vi "Dresden R2R Sputter 03.02.2018 IY24.vi"() -> ()   [LabVIEW 2009] (continued)
                                }
                                }
                                }
                                }
                                }
                                frame #1 {
                                }
                                }
                                }
                                frame #1 {
                                }
                                }
                                }
                                }
                                }
                                frame #1 {
                                }
                                }
                                }
                                frame #1 {
                                n26473 = local read "Semi"() -> (w31686:bool)
                                n26474 = case shown="False" w31686 {
                                frame #0 {
                                n26475 = Wait (ms)(milliseconds to wait=u32 1000) -> ()  [unwired: 1 out]
                                n26476 = local write "SDC1 29"(TRUE ("SDC1 29")) -> ()
                                }
                                frame #1 {
                                }
                                }
                                }
                                }
                                }
                                frame #27 {
                                n26477 = local read "Semi"() -> (w31689:bool)
                                n26478 = case shown="False" w31689 {
                                frame #0 {
                                n26479 = local write "Cnt_Do_Buzzer"(TRUE ("SDC1 30")) -> ()
                                n26480 = Wait (ms)(milliseconds to wait=u32 2500) -> ()  [unwired: 1 out]
                                n26481 = local write "SDC1 30"(TRUE ("SDC1 30")) -> ()
                                }
                                frame #1 {
                                }
                                }
                                }
                                frame #28 {
                                n26482 = local read "Semi"() -> (w31693:bool)
                                n26483 = case shown="False" w31693 {
                                frame #0 {
                                n26484 = local write "Cnt_Do_Buzzer"(FALSE ("SDC1 30")) -> ()
                                n26485 = Wait (ms)(milliseconds to wait=u32 1000) -> ()  [unwired: 1 out]
                                }
                                frame #1 {
                                }
                                }
                                }
                                }
                                }
                                frame #1 {
                                }
                                }
                                }
                              }
                            }
                            frame #1 {
                              n26486 = local read "Single_ch3_Interlock"() -> (w31696:dbl)
                              n26487 = local read "Ch3_pressure"() -> (w31700:dbl)
                              n26488 = local read "started_up_ch3"() -> (w31698:bool)
                              n26489 = In Range and Coerce(upper limit=w31696, x=w31700, lower limit=1e-08) -> (In Range?=w31701:bool)  [unwired: 1 out]
                              n26490 = And(x=w31701, y=w31698) -> (x .and. y?=w31697:bool)
                              n26491 = case shown="True" w31697 {
                                frame #0 {
                                }
                                frame #1 {
                                n26492 = local read "Semi"() -> (w31702:bool)
                                n26493 = case shown="False" w31702 {
                                frame #0 {
                                n26494 = stacked-sequence {
                                frame #0 {
                                n26495 = stacked-sequence {
                                frame #0 {
                                n26496 = local read "Semi"() -> (w31703:bool)
                                n26497 = case shown="False" w31703 {
                                frame #0 {
                                w31707 = FALSE ("Casette_servo_start/stop_do")
                                n26498 = local write "Ch3_Sov_Ar_do"(FALSE ("Ch1_Sov_Ar_do")) -> ()
                                n26499 = local write "Ar_auto_set_zero_ch3"(TRUE ("Dc_auto_set_zero")) -> ()
                                n26500 = local write "Dc_host_auto"(TRUE ("Dc_host_auto")) -> ()
                                n26501 = local write "final_process_messages"("Coating was Completed" ("final_process_messages")) -> ()
                                n26502 = local write "system_status"("Coating Mode is Active" ("system_status")) -> ()
                                n26503 = local write "Casette_servo_start/stop_do"(w31707) -> ()
                                n26504 = local write "Tension_controllers_start/stop_do"(w31707) -> ()
                                n26505 = local write "Cnt_Dcps_sw1_do"(FALSE ("Cnt_Dcps_sw1_do")) -> ()
                                }
                                frame #1 {
                                }
                                }
                                }
                                frame #1 {
                                n26506 = local read "Semi"() -> (w31711:bool)
                                n26507 = case shown="False" w31711 {
                                frame #0 {
                                n26508 = Wait (ms)(milliseconds to wait=u32 2500) -> ()  [unwired: 1 out]
                                }
                                frame #1 {
                                }
                                }
                                }
                                frame #2 {
                                n26509 = local read "Semi"() -> (w31713:bool)
                                n26510 = case shown="False" w31713 {
                                frame #0 {
                                n26511 = local write "Ch2_SRV_start_stop_do"(FALSE ("Ch1_SRV_start_stop_do")) -> ()
                                }
                                frame #1 {
                                }
                                }
                                }
                                frame #3 {
                                n26512 = local read "Semi"() -> (w31715:bool)
                                n26513 = case shown="False" w31715 {
                                frame #0 {
                                n26514 = Wait (ms)(milliseconds to wait=u32 2500) -> ()  [unwired: 1 out]
                                }
                                frame #1 {
                                }
                                }
                                }
                                frame #4 {
                                n26515 = local read "Semi"() -> (w31717:bool)
                                n26516 = case shown="False" w31717 {
                                frame #0 {
                                n26517 = Wait (ms)(milliseconds to wait=u32 1000) -> ()  [unwired: 1 out]
                                n26518 = local write "SDC1 1"(TRUE ("CMW1")) -> ()
                                }
                                frame #1 {
                                }
                                }
                                }
                                }
                                }
                                frame #1 {
                                n26519 = local read "ch_present_position"() -> (w31722:dbl)
                                n26520 = Not Equal?(x=w31722, y=3.0) -> (x != y?=w31720:bool)
                                n26521 = case shown="True" w31720 {
                                frame #0 {
                                }
                                frame #1 {
                                n26522 = stacked-sequence {
                                frame #0 {
                                n26523 = local write "Set chamber"(3.0 ("Set chamber")) -> ()
                                n26524 = Wait (ms)(milliseconds to wait=u32 100) -> ()  [unwired: 1 out]
                                }
                                frame #1 {
                                n26525 = local write "Auto_set_transfer"(TRUE ("Auto_set_transfer")) -> ()
                                }
                                frame #2 {
                                n26526 = while {
                                stop <- w31727 stop-if-true
                                n26527 = Wait Until Next ms Multiple(millisecond multiple=u32 300) -> ()  [unwired: 1 out]
                                n26528 = local read "Auto_set_transfer"() -> (w31728:bool)
                                n26529 = local read "Semi"() -> (w31730:bool)
                                n26530 = Not(x=w31728) -> (.not. x?=w31729:bool)
                                n26531 = Or(x=w31729, y=w31730) -> (x .or. y?=w31727:bool)
                                }
                                }
                                frame #3 {
                                n26532 = Wait (ms)(milliseconds to wait=u32 300) -> ()  [unwired: 1 out]
                                n26533 = local write "SDC2 19"(TRUE ("SMW1 2")) -> ()
                                }
                                }
                                }
                                }
                                }
                                frame #2 {
                                # "WATER FLOW CONTROL OPEN"
                                n26534 = stacked-sequence {
                                frame #0 {
                                n26535 = local read "Semi"() -> (w31733:bool)
                                n26536 = case shown="False" w31733 {
                                frame #0 {
                                n26537 = while {
                                i -> [w31739]
                                stop <- w31734 stop-if-true
                                n26538 = Greater?(x=w31739, y=100) -> (0:w31738:bool)
                                n26539 = case shown="True" w31738 {
                                frame #0 {
                                }
                                frame #1 {
                                n26540 = local write "Semi"(TRUE ("Semi")) -> ()
                                n26541 = local write "Error Message"("Coating Process  \nwas cancelled.\nPlease check water \nflow connection." ("Error Message")) -> ()
                                }
                                }
                                n26542 = local read "Ch4_WFS_di"() -> (w31737:bool)
                                n26543 = case shown="True" w31737 {
                                tunnel: [TRUE FALSE] -> w31736
                                frame #0 {
                                }
                                frame #1 {
                                n26544 = local write "Ch4_WFC_do"(FALSE ("Ch1_WFC_do")) -> ()
                                n26545 = Wait Until Next ms Multiple(millisecond multiple=u32 200) -> ()  [unwired: 1 out]
                                }
                                }
                                n26546 = local read "Semi"() -> (w31735:bool)
                                n26547 = Or(x=w31736, y=w31735) -> (x .or. y?=w31734:bool)
                                }
                                }
                                frame #1 {
                                }
                                }
                                }
                                frame #1 {
                                n26548 = local read "Semi"() -> (w31747:bool)
                                n26549 = case shown="False" w31747 {
                                frame #0 {
                                n26550 = while {
                                i -> [w31753]
                                stop <- w31748 stop-if-true
                                n26551 = Greater?(x=w31753, y=100) -> (0:w31752:bool)
                                n26552 = case shown="True" w31752 {
                                frame #0 {
                                }
                                frame #1 {
                                n26553 = local write "Semi"(TRUE ("Semi")) -> ()
                                n26554 = local write "Error Message"("Coating Process  \nwas cancelled.\nPlease check water \nflow connection." ("Error Message")) -> ()
                                }
                                }
                                n26555 = local read "Ch1_WFS_di"() -> (w31751:bool)
                                n26556 = case shown="True" w31751 {
                                tunnel: [TRUE FALSE] -> w31750
                                frame #0 {
                                }
                                frame #1 {
                                n26557 = local write "Ch1_WFC_do"(FALSE ("Ch1_WFC_do")) -> ()
                                n26558 = Wait Until Next ms Multiple(millisecond multiple=u32 200) -> ()  [unwired: 1 out]
                                }
                                }
                                n26559 = local read "Semi"() -> (w31749:bool)
                                n26560 = Or(x=w31750, y=w31749) -> (x .or. y?=w31748:bool)
                                }
                                }
                                frame #1 {
                                }
                                }
                                }
                                frame #2 {
                                n26561 = local read "Semi"() -> (w31761:bool)
                                n26562 = case shown="False" w31761 {
                                frame #0 {
                                n26563 = while {
                                i -> [w31767]
                                stop <- w31762 stop-if-true
                                n26564 = Greater?(x=w31767, y=100) -> (0:w31766:bool)
                                n26565 = case shown="True" w31766 {
                                frame #0 {
                                }
                                frame #1 {
                                n26566 = local write "Semi"(TRUE ("Semi")) -> ()
                                n26567 = local write "Error Message"("Coating Process  \nwas cancelled.\nPlease check water \nflow connection." ("Error Message")) -> ()
                                }
                                }
                                n26568 = local read "Ch2_WFS_di"() -> (w31765:bool)
                                n26569 = case shown="True" w31765 {
                                tunnel: [TRUE FALSE] -> w31764
                                frame #0 {
                                }
                                frame #1 {
                                n26570 = local write "Ch2_WFC_do"(FALSE ("Ch1_WFC_do")) -> ()
                                n26571 = Wait Until Next ms Multiple(millisecond multiple=u32 200) -> ()  [unwired: 1 out]
                                }
                                }
                                n26572 = local read "Semi"() -> (w31763:bool)
                                n26573 = Or(x=w31764, y=w31763) -> (x .or. y?=w31762:bool)
                                }
                                }
                                frame #1 {
                                }
                                }
                                }
                                frame #3 {
                                n26574 = local read "Semi"() -> (w31775:bool)
                                n26575 = case shown="False" w31775 {
                                frame #0 {
                                n26576 = local write "SDC1 2"(TRUE ("SDC1 2")) -> ()
                                n26577 = Wait (ms)(milliseconds to wait=u32 1000) -> ()  [unwired: 1 out]
                                }
                                frame #1 {
                                }
                                }
                                }
                                frame #4 {
                                n26578 = local read "Semi"() -> (w31778:bool)
                                n26579 = case shown="False" w31778 {
                                frame #0 {
                                n26580 = while {
                                i -> [w31784]
                                stop <- w31779 stop-if-true
                                n26581 = Greater?(x=w31784, y=100) -> (0:w31783:bool)
                                n26582 = case shown="True" w31783 {
                                frame #0 {
                                }
                                frame #1 {
                                n26583 = local write "Semi"(TRUE ("Semi")) -> ()
                                n26584 = local write "Error Message"("Coating Process  \nwas cancelled.\nPlease check water \nflow connection." ("Error Message")) -> ()
                                }
                                }
                                n26585 = local read "Ch3_WFS_di"() -> (w31782:bool)
                                n26586 = case shown="False" w31782 {
                                tunnel: [FALSE TRUE] -> w31781
                                frame #0 {
                                n26587 = local write "Ch3_WFC_do"(TRUE ("Ch1_WFC_do")) -> ()
                                n26588 = Wait Until Next ms Multiple(millisecond multiple=u32 200) -> ()  [unwired: 1 out]
                                }
                                frame #1 {
                                }
                                }
                                n26589 = local read "Semi"() -> (w31780:bool)
                                n26590 = Or(x=w31781, y=w31780) -> (x .or. y?=w31779:bool)
                                }
                                }
                                frame #1 {
                                }
                                }
                                }
                                }
                                }
                                frame #3 {
                                # "BG-BV open"
                                n26591 = stacked-sequence {
                                frame #0 {
                                n26592 = local read "Semi"() -> (w31792:bool)
                                n26593 = case shown="False" w31792 {
                                frame #0 {
                                n26594 = while {
                                i -> [w31798]
                                stop <- w31793 stop-if-true
                                n26595 = Greater?(x=w31798, y=50) -> (0:w31797:bool)
                                n26596 = case shown="True" w31797 {
                                frame #0 {
                                }
                                frame #1 {
                                n26597 = local write "Semi"(TRUE ("Semi")) -> ()
                                n26598 = local write "Error Message"("Coating Process  \nwas cancelled.\nPlease check \nBG-BV connection." ("Error Message")) -> ()
                                }
                                }
                                n26599 = local read "Ch3_Bg_bv_di"() -> (w31796:bool)
                                n26600 = case shown="False" w31796 {
                                tunnel: [FALSE TRUE] -> w31795
                                frame #0 {
                                n26601 = local write "Ch3_Bg_bv_do"(TRUE ("Ch1_WFC_do")) -> ()
                                n26602 = Wait Until Next ms Multiple(millisecond multiple=u32 200) -> ()  [unwired: 1 out]
                                }
                                frame #1 {
                                }
                                }
                                n26603 = local read "Semi"() -> (w31794:bool)
                                n26604 = Or(x=w31795, y=w31794) -> (x .or. y?=w31793:bool)
                                }
                                }
                                frame #1 {
                                }
                                }
                                }
                                frame #1 {
                                n26605 = local read "Semi"() -> (w31806:bool)
                                n26606 = case shown="False" w31806 {
                                frame #0 {
                                n26607 = Wait (ms)(milliseconds to wait=u32 1000) -> ()  [unwired: 1 out]
                                n26608 = local write "SDC1 4"(TRUE ("SDC1 4")) -> ()
                                }
                                frame #1 {
                                }
                                }
                                }
                                }
                                }
                                frame #4 {
                                # "Baratron set zero"
                                n26609 = stacked-sequence {
                                frame #0 {
                                n26610 = local write "Pc_bv3_auto_baratron_set_zero"(TRUE ("Pc_bv2_auto_baratron_set_zero")) -> ()
                                }
                                frame #1 {
                                n26611 = while {
                                i -> [w31814]
                                stop <- w31811 stop-if-true
                                n26612 = Greater?(x=w31814, y=50 ("Baratron set zero time 2")) -> (0:w31813:bool)
                                n26613 = case shown="True" w31813 {
                                frame #0 {
                                }
                                frame #1 {
                                n26614 = local write "Semi"(TRUE ("Semi")) -> ()
                                n26615 = local write "Error Message"("" ("Error Message")) -> ()
                                }
                                }
                                n26616 = local read "Pressure_ch3"() -> (w31810:i32)
                                n26617 = Less?(x=w31810, y=0.1 ("Pressure Check for baratron set zero")) -> (x < y?=w31817:bool)
                                n26618 = case shown="False" w31817 {
                                tunnel: [FALSE TRUE] -> w31816
                                frame #0 {
                                n26619 = Wait Until Next ms Multiple(millisecond multiple=u32 200) -> ()  [unwired: 1 out]
                                }
                                frame #1 {
                                }
                                }
                                n26620 = local read "Semi"() -> (w31815:bool)
                                n26621 = Or(x=w31816, y=w31815) -> (x .or. y?=w31811:bool)
                                }
                                }
                                frame #2 {
                                n26622 = local read "Semi"() -> (w31824:bool)
                                n26623 = case shown="False" w31824 {
                                frame #0 {
                                n26624 = local write "SDC1 2b"(TRUE ("SDC1 2b")) -> ()
                                n26625 = Wait (ms)(milliseconds to wait=u32 1000) -> ()  [unwired: 1 out]
                                }
                                frame #1 {
                                }
                                }
                                }
                                }
                                }
                                frame #5 {
                                # "CC CLOSE"
                                n26626 = stacked-sequence {
                                frame #0 {
                                n26627 = local read "Semi"() -> (w31827:bool)
                                n26628 = case shown="False" w31827 {
                                frame #0 {
                                n26629 = while {
                                i -> [w31833]
                                stop <- w31828 stop-if-true
                                n26630 = Greater?(x=w31833, y=50) -> (0:w31832:bool)
                                n26631 = case shown="True" w31832 {
                                frame #0 {
                                }
                                frame #1 {
                                n26632 = local write "Semi"(TRUE ("Semi")) -> ()
                                n26633 = local write "Error Message"("Coating Process  \nwas cancelled.\nPlease check \nBG-BV connection." ("Error Message")) -> ()
                                }
                                }
                                n26634 = local read "Ch3_Cc_on_off_di"() -> (w31831:bool)
                                n26635 = case shown="True" w31831 {
                                tunnel: [TRUE FALSE] -> w31830
                                frame #0 {
                                }
                                frame #1 {
                                n26636 = local write "Ch3_Cc_on_off_do"(FALSE ("Ch1_WFC_do")) -> ()
                                n26637 = Wait Until Next ms Multiple(millisecond multiple=u32 200) -> ()  [unwired: 1 out]
                                }
                                }
                                n26638 = local read "Semi"() -> (w31829:bool)
                                n26639 = Or(x=w31830, y=w31829) -> (x .or. y?=w31828:bool)
                                }
                                }
                                frame #1 {
                                }
                                }
                                }
                                frame #1 {
                                n26640 = local read "Semi"() -> (w31841:bool)
                                n26641 = case shown="False" w31841 {
                                frame #0 {
                                n26642 = local write "SDC1 3"(TRUE ("SDC1 3")) -> ()
                                n26643 = Wait (ms)(milliseconds to wait=u32 1000) -> ()  [unwired: 1 out]
                                }
                                frame #1 {
                                }
                                }
                                }
                                }
                                }
                                frame #6 {
                                # "PC-BV CLOSE"
                                n26644 = stacked-sequence {
                                frame #0 {
                                n26645 = local read "Semi"() -> (w31844:bool)
                                n26646 = case shown="False" w31844 {
                                frame #0 {
                                n26647 = stacked-sequence {
                                frame #0 {
                                n26648 = local read "Semi"() -> (w31845:bool)
                                n26649 = case shown="False" w31845 {
                                frame #0 {
                                n26650 = local write "Pc_bv3_auto_close"(TRUE ("Tp1_auto_start")) -> ()
                                }
                                frame #1 {
                                }
                                }
                                }
                                frame #1 {
                                n26651 = local read "Semi"() -> (w31847:bool)
                                n26652 = case shown="False" w31847 {
                                frame #0 {
                                n26653 = Wait (ms)(milliseconds to wait=u32 1000) -> ()  [unwired: 1 out]
                                }
                                frame #1 {
                                }
                                }
                                }
                                frame #2 {
                                n26654 = local read "Semi"() -> (w31849:bool)
                                n26655 = case shown="False" w31849 {
                                frame #0 {
                                n26656 = while {
                                i -> [w31855]
                                stop <- w31851 stop-if-true
                                n26657 = local read "Pc_bv_closed_ch3"() -> (w31853:bool)
                                n26658 = Greater?(x=w31855, y=120) -> (0:w31854:bool)
                                n26659 = local read "Semi"() -> (w31852:bool)
                                n26660 = Compound Arithmetic op=OR(w31852, w31853, w31854) -> (w31851:bool)
                                n26661 = Wait (ms)(milliseconds to wait=u32 500) -> ()  [unwired: 1 out]
                                }
                                }
                                frame #1 {
                                }
                                }
                                }
                                frame #3 {
                                n26662 = local read "Semi"() -> (w31857:bool)
                                n26663 = case shown="False" w31857 {
                                frame #0 {
                                n26664 = local read "Pc_bv_closed_ch3"() -> (w31858:bool)
                                n26665 = case shown="False" w31858 {
                                frame #0 {
                                n26666 = local write "Pc_bv3_auto_close"(TRUE ("Pc_bv1_auto_open")) -> ()
                                }
                                frame #1 {
                                }
                                }
                                }
                                frame #1 {
                                }
                                }
                                }
                                frame #4 {
                                n26667 = local read "Semi"() -> (w31860:bool)
                                n26668 = case shown="False" w31860 {
                                frame #0 {
                                n26669 = local read "Pc_bv_closed_ch3"() -> (w31861:bool)
                                n26670 = case shown="False" w31861 {
                                frame #0 {
                                n26671 = Wait (ms)(milliseconds to wait=u32 1000) -> ()  [unwired: 1 out]
                                }
                                frame #1 {
                                }
                                }
                                }
                                frame #1 {
                                }
                                }
                                }
                                frame #5 {
                                n26672 = local read "Semi"() -> (w31863:bool)
                                n26673 = case shown="False" w31863 {
                                frame #0 {
                                n26674 = while {
                                i -> [w31869]
                                stop <- w31865 stop-if-true
                                n26675 = local read "Pc_bv_closed_ch3"() -> (w31867:bool)
                                n26676 = Greater?(x=w31869, y=120) -> (0:w31868:bool)
                                n26677 = local read "Semi"() -> (w31866:bool)
                                n26678 = Compound Arithmetic op=OR(w31866, w31867, w31868) -> (w31865:bool)
                                n26679 = Wait (ms)(milliseconds to wait=u32 500) -> ()  [unwired: 1 out]
                                }
                                }
                                frame #1 {
                                }
                                }
                                }
                                frame #6 {
                                n26680 = local read "Semi"() -> (w31871:bool)
                                n26681 = case shown="False" w31871 {
                                frame #0 {
                                n26682 = local read "Pc_bv_closed_ch3"() -> (w31872:bool)
                                n26683 = case shown="False" w31872 {
                                frame #0 {
                                n26684 = local write "Error Message"("Start up process  cancelled\nbecause  PC-BV not closed.\nPlease check PC-BV1 connections." ("Error Message")) -> ()
                                n26685 = Wait (ms)(milliseconds to wait=u32 1000) -> ()  [unwired: 1 out]
                                }
                                frame #1 {
                                }
                                }
                                }
                                frame #1 {
                                }
                                }
                                }
                                }
                                }
                                frame #1 {
                                }
                                }
                                }
                                frame #1 {
                                n26686 = local read "Semi"() -> (w31875:bool)
                                n26687 = case shown="False" w31875 {
                                frame #0 {
                                n26688 = local write "SDC1 5"(TRUE ("SDC1 5")) -> ()
                                n26689 = Wait (ms)(milliseconds to wait=u32 1000) -> ()  [unwired: 1 out]
                                }
                                frame #1 {
                                }
                                }
                                }
                                }
                                }
                                frame #7 {
                                # "SOV-AR OPEN"
                                n26690 = stacked-sequence {
                                frame #0 {
                                n26691 = local read "Semi"() -> (w31878:bool)
                                n26692 = case shown="False" w31878 {
                                frame #0 {
                                n26693 = while {
                                i -> [w31884]
                                stop <- w31879 stop-if-true
                                n26694 = Greater?(x=w31884, y=50) -> (0:w31883:bool)
                                n26695 = case shown="True" w31883 {
                                frame #0 {
                                }
                                frame #1 {
                                n26696 = local write "Semi"(TRUE ("Semi")) -> ()
                                n26697 = local write "Error Message"("Coating Process  \nwas cancelled.\nPlease check \nSOV-Ar connection." ("Error Message")) -> ()
                                }
                                }
                                n26698 = local read "Ch3_Sov_Ar_di"() -> (w31882:bool)
                                n26699 = case shown="False" w31882 {
                                tunnel: [FALSE TRUE] -> w31881
                                frame #0 {
                                n26700 = local write "Ch3_Sov_Ar_do"(TRUE ("Ch1_WFC_do")) -> ()
                                n26701 = Wait Until Next ms Multiple(millisecond multiple=u32 200) -> ()  [unwired: 1 out]
                                }
                                frame #1 {
                                }
                                }
                                n26702 = local read "Semi"() -> (w31880:bool)
                                n26703 = Or(x=w31881, y=w31880) -> (x .or. y?=w31879:bool)
                                }
                                }
                                frame #1 {
                                }
                                }
                                }
                                frame #1 {
                                n26704 = local read "Semi"() -> (w31892:bool)
                                n26705 = case shown="False" w31892 {
                                frame #0 {
                                n26706 = while {
                                i -> [w31897]
                                stop <- w31895 stop-if-true
                                n26707 = Greater?(x=w31897, y=5) -> (0:w31893:bool)
                                n26708 = Wait Until Next ms Multiple(millisecond multiple=u32 1000) -> ()  [unwired: 1 out]
                                n26709 = local read "Semi"() -> (w31896:bool)
                                n26710 = Or(x=w31893, y=w31896) -> (x .or. y?=w31895:bool)
                                }
                                }
                                frame #1 {
                                }
                                }
                                }
                                frame #2 {
                                n26711 = local read "Semi"() -> (w31899:bool)
                                n26712 = case shown="False" w31899 {
                                frame #0 {
                                n26713 = local write "SDC1 6"(TRUE ("SDC1 6")) -> ()
                                n26714 = Wait (ms)(milliseconds to wait=u32 1000) -> ()  [unwired: 1 out]
                                }
                                frame #1 {
                                }
                                }
                                }
                                }
                                }
                                frame #8 {
                                # "CHECK CHAMBER PRESSURE"
                                n26715 = stacked-sequence {
                                frame #0 {
                                n26716 = local read "Semi"() -> (w31902:bool)
                                n26717 = case shown="False" w31902 {
                                frame #0 {
                                n26718 = while {
                                i -> [w31910]
                                stop <- w31904 stop-if-true
                                n26719 = Greater?(x=w31910, y=300) -> (0:w31909:bool)
                                n26720 = case shown="True" w31909 {
                                frame #0 {
                                }
                                frame #1 {
                                n26721 = local write "Semi"(TRUE ("Semi")) -> ()
                                n26722 = local write "Error Message"("Coating Process cancelled.\nPlease check chamber \nconnections." ("Error Message")) -> ()
                                }
                                }
                                n26723 = local read "Ch_pg_press_ch3_gui"() -> (w31903:dbl)
                                n26724 = Greater Or Equal?(x=w31903, y=0.9 ("CHAMBER PRESSURE 4")) -> (x >= y?=w31907:bool)
                                n26725 = case shown="True" w31907 {
                                tunnel: [TRUE FALSE] -> w31906
                                frame #0 {
                                }
                                frame #1 {
                                n26726 = Wait Until Next ms Multiple(millisecond multiple=u32 200) -> ()  [unwired: 1 out]
                                }
                                }
                                n26727 = local read "Semi"() -> (w31905:bool)
                                n26728 = Or(x=w31906, y=w31905) -> (x .or. y?=w31904:bool)
                                }
                                }
                                frame #1 {
                                }
                                }
                                }
                                frame #1 {
                                n26729 = local read "Semi"() -> (w31917:bool)
                                n26730 = case shown="False" w31917 {
                                frame #0 {
                                n26731 = Wait (ms)(milliseconds to wait=u32 1000) -> ()  [unwired: 1 out]
                                n26732 = local write "SDC1 8"(TRUE ("SDC1 8")) -> ()
                                }
                                frame #1 {
                                }
                                }
                                }
                                }
                                }
                                frame #9 {
                                # "PC-BV OPEN"
                                n26733 = stacked-sequence {
                                frame #0 {
                                n26734 = local read "Semi"() -> (w31920:bool)
                                n26735 = case shown="False" w31920 {
                                frame #0 {
                                n26736 = stacked-sequence {
                                frame #0 {
                                n26737 = local read "Semi"() -> (w31921:bool)
                                n26738 = case shown="False" w31921 {
                                frame #0 {
                                n26739 = local write "Pc_bv3_auto_open"(TRUE ("Tp1_auto_start")) -> ()
                                }
                                frame #1 {
                                }
                                }
                                }
                                frame #1 {
                                n26740 = local read "Semi"() -> (w31923:bool)
                                n26741 = case shown="False" w31923 {
                                frame #0 {
                                n26742 = Wait (ms)(milliseconds to wait=u32 1000) -> ()  [unwired: 1 out]
                                }
                                frame #1 {
                                }
                                }
                                }
                                frame #2 {
                                n26743 = local read "Semi"() -> (w31925:bool)
                                n26744 = case shown="False" w31925 {
                                frame #0 {
                                n26745 = while {
                                i -> [w31931]
                                stop <- w31927 stop-if-true
                                n26746 = local read "Pc_bv_opened_ch3"() -> (w31929:bool)
                                n26747 = Greater?(x=w31931, y=120) -> (0:w31930:bool)
                                n26748 = local read "Semi"() -> (w31928:bool)
                                n26749 = Compound Arithmetic op=OR(w31928, w31929, w31930) -> (w31927:bool)
                                n26750 = Wait (ms)(milliseconds to wait=u32 500) -> ()  [unwired: 1 out]
                                }
                                }
                                frame #1 {
                                }
                                }
                                }
                                frame #3 {
                                n26751 = local read "Semi"() -> (w31933:bool)
                                n26752 = case shown="False" w31933 {
                                frame #0 {
                                n26753 = local read "Pc_bv_opened_ch3"() -> (w31934:bool)
                                n26754 = case shown="False" w31934 {
                                frame #0 {
                                n26755 = local write "Pc_bv3_auto_open"(TRUE ("Pc_bv1_auto_open")) -> ()
                                }
                                frame #1 {
                                }
                                }
                                }
                                frame #1 {
                                }
                                }
                                }
                                frame #4 {
                                n26756 = local read "Semi"() -> (w31936:bool)
                                n26757 = case shown="False" w31936 {
                                frame #0 {
                                n26758 = local read "Pc_bv_opened_ch3"() -> (w31937:bool)
                                n26759 = case shown="False" w31937 {
                                frame #0 {
                                n26760 = Wait (ms)(milliseconds to wait=u32 1000) -> ()  [unwired: 1 out]
                                }
                                frame #1 {
                                }
                                }
                                }
                                frame #1 {
                                }
                                }
                                }
                                frame #5 {
                                n26761 = local read "Semi"() -> (w31939:bool)
                                n26762 = case shown="False" w31939 {